vi "Login.vi"() -> ()   [LabVIEW 2020]
uses:
  System.Windows.Forms
  Global_Variable/Global.vi
  <userlib>/_MGI/Menu Building/MenuItemStatusChange/MGI_MenuItemStatusChange.lvclass
panel:
  in  "枚举":enum16{"左工位", "右工位"}(ring)
  in  "菜单":refnum<k24>(container)
  in  "联机模式":enum16{"单机", "追溯"}(ring)
  in  "登陆":bool
  in  "密   码":string
  in  "用户名":string
  out "数据库连接成功":bool
  # "传感器对中台"
  # "数据库状态"
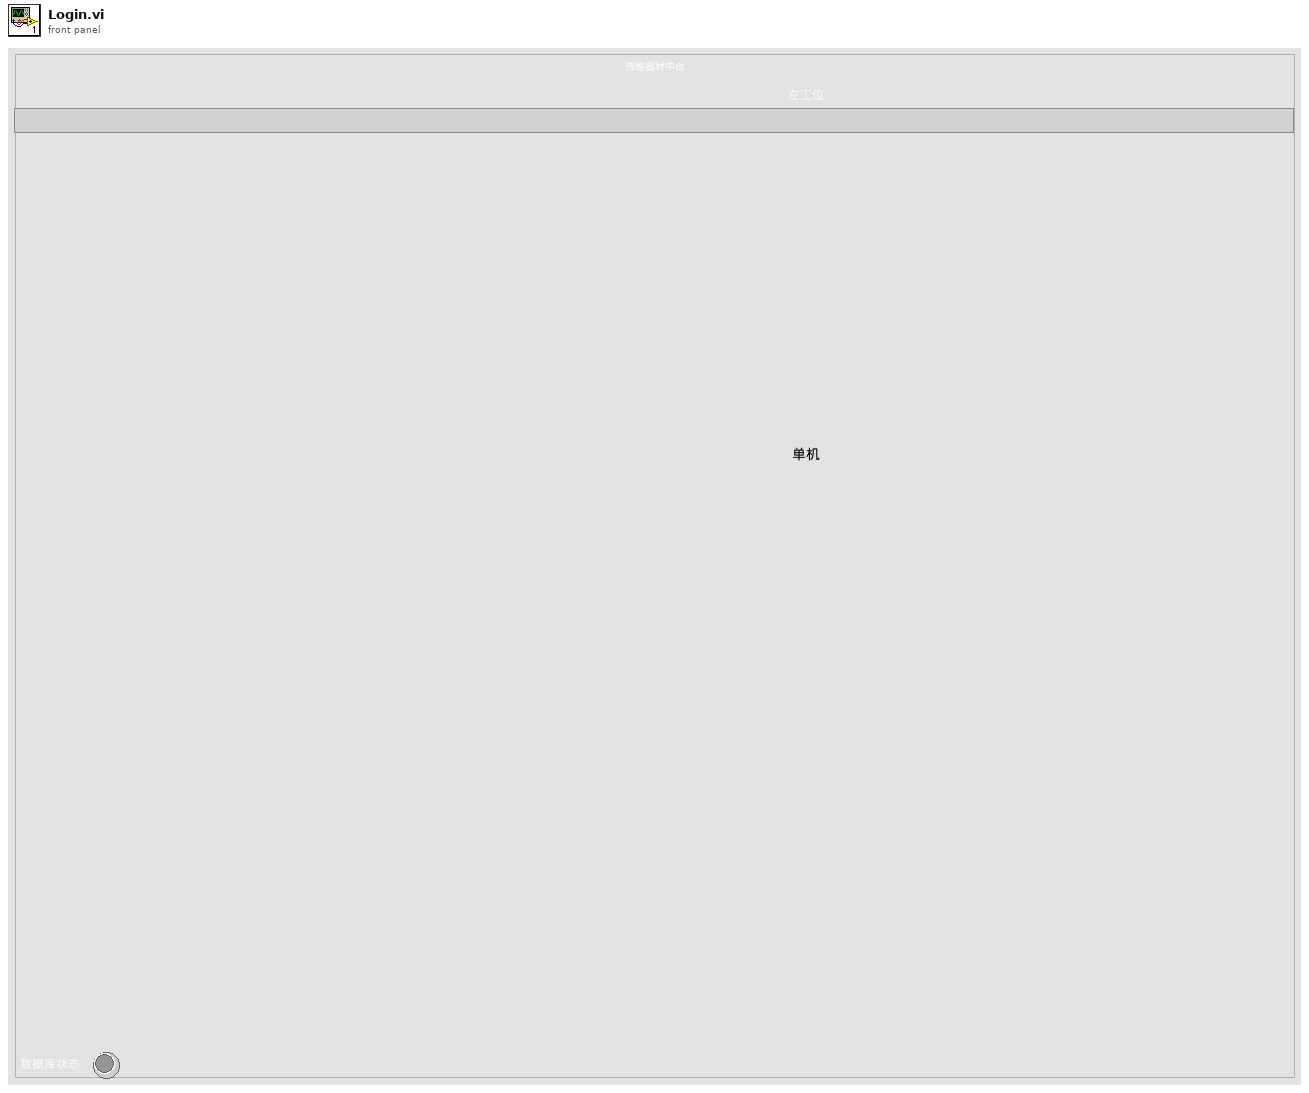
[diagram p1: front panel]
types:
  T1 = enum8{"Enabled", "Disabled", "Disabled and Grayed Out"}
  T2 = enum32{"Invalid", "Standard", "Closed", "Hidden", "Minimized", "Maximized"}
  T3 = cluster{"data[0]":string, "data[1]":string, "data[2]":string, "data[3]":string}
  T4 = typedef "eventvkey.ctl" = enum16{"ASCII", "Enter", "Return", "Shift", "Ctrl", "Alt", "Cmd", "Opt", "Caps", "NumLock", "Clear", "Break", "Up", "Down", "Left", "Right", "Insert", "Delete", "Home", "End", "PageUp", "PageDown", "Escape", "Help", "Pause", "ScrollLock", "F1", "F2", "F3", "F4", "F5", "F6", "F7", "F8", "F9", "F10", "F11", "F12", "F13", "F14", "F15", "F16", "F17", "F18", "F19", "F20", "F21", "F22", "F23", "F24", "Play", "VolumeUp", "VolumeDown", "Mute", "Two Byte Char"}
  T5 = cluster{"用户编号":string, "用户名":string, "用户密码(密文)":string, "用户权限":string}
  T6 = cluster{"操作员编号":string, "操作员姓名":string, "操作员权限":string, "联机模式":enum16{"单机", "追溯"}}
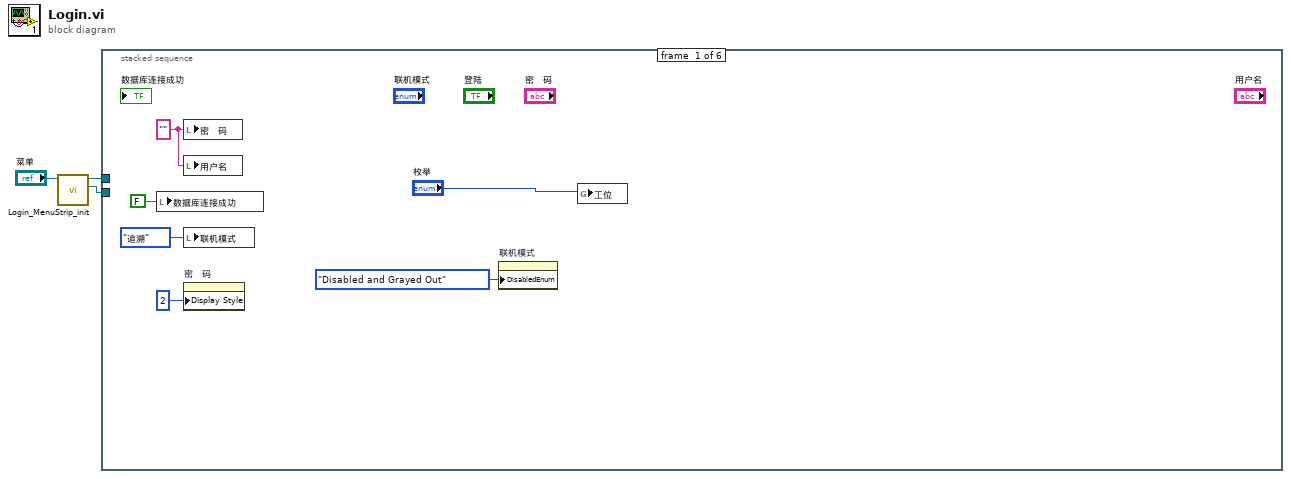
[diagram p0: block diagram]
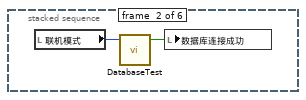
[diagram p2: hidden frame]
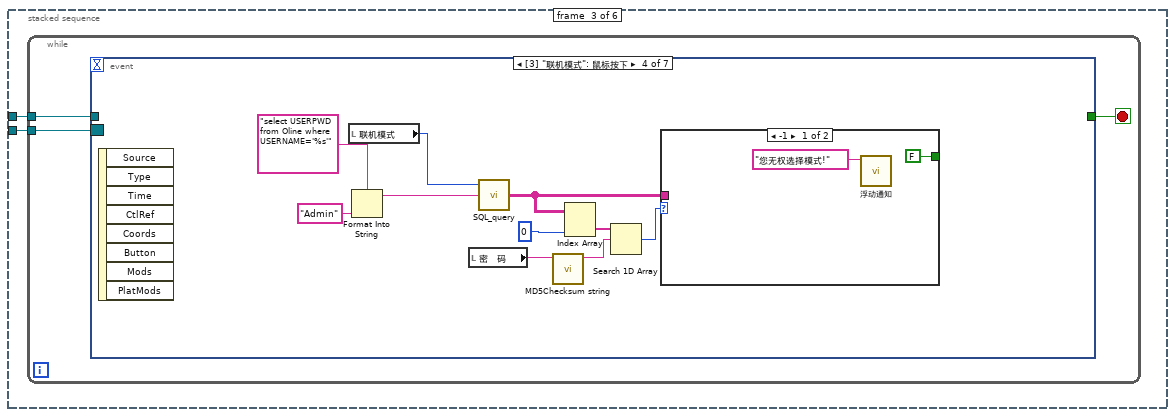
[diagram p3: hidden frame]
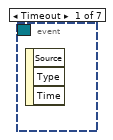
[diagram p4: hidden frame]
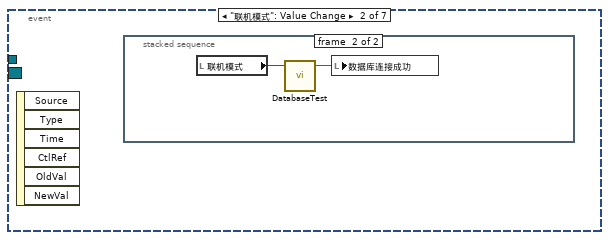
[diagram p5: hidden frame]
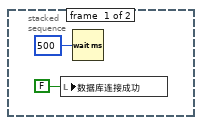
[diagram p6: hidden frame]
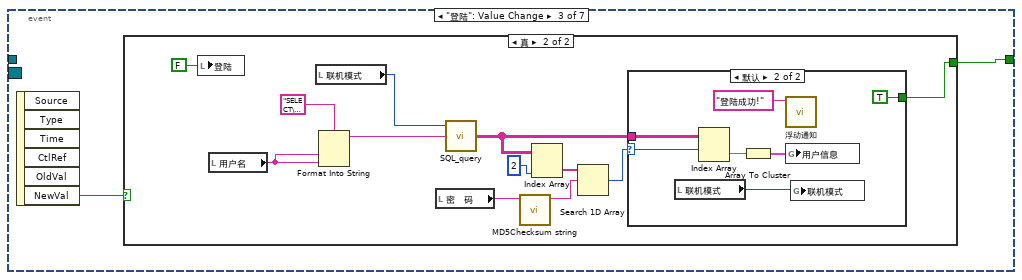
[diagram p7: hidden frame]
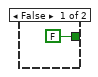
[diagram p8: hidden frame]
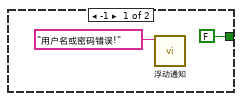
[diagram p9: hidden frame]
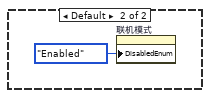
[diagram p10: hidden frame]
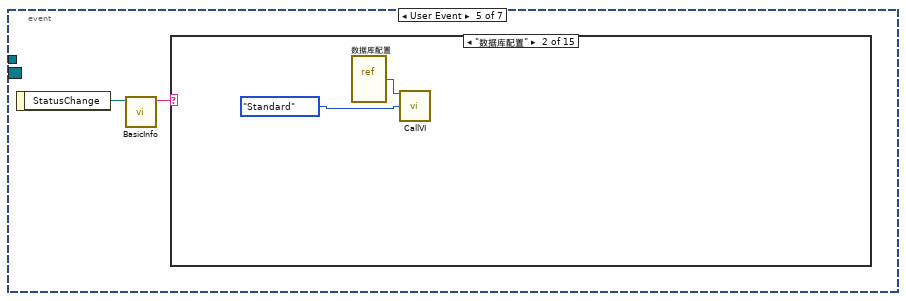
[diagram p11: hidden frame]
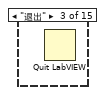
[diagram p13: hidden frame]
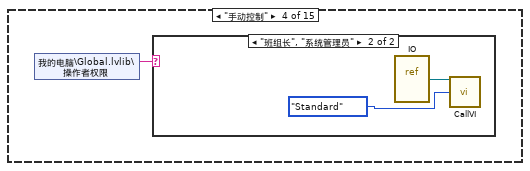
[diagram p14: hidden frame]
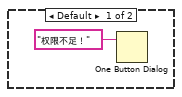
[diagram p15: hidden frame]
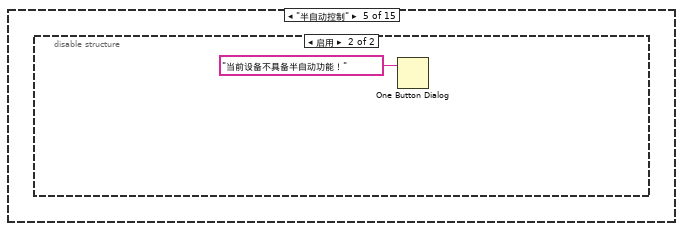
[diagram p16: hidden frame]
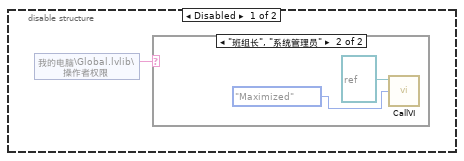
[diagram p17: hidden frame]
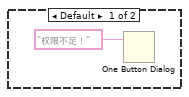
[diagram p18: hidden frame]
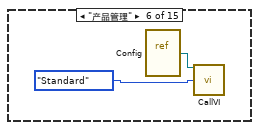
[diagram p19: hidden frame]
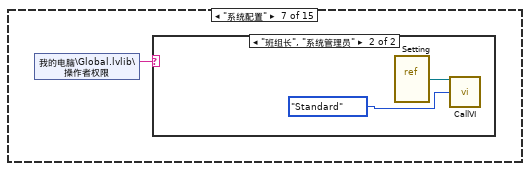
[diagram p20: hidden frame]
diagram:
  n1 = call "Login_MenuStrip_init.vi"("MenuStrip"="菜单") -> ("MenuStrip_Event"=w2:refnum<event-registration>, "Menu out"=w1:refnum<class "MGI_MenuStrip.lvclass">)  [unwired: 9 in]
  n2 = stacked-sequence {
    tunnel: w2 -> [_ _ w13 _ _ _]
    tunnel: w1 -> [_ _ w12 _ _ _]
    frame #0 {
      w8 = ""
      n3 = local write "数据库连接成功"(FALSE ("数据库连接成功")) -> ()
      n4 = local write "密   码"(w8) -> ()
      n5 = local write "用户名"(w8) -> ()
      n6 = local write "联机模式"(enum16{"单机", "追溯"}."追溯" ("联机模式")) -> ()
      n7 = property on="密   码" class="Str"("Display Style"=u32 2 ("显示样式")) -> ()  [unwired: 2 in, 2 out]
      n8 = property on="联机模式" class="Enum (严格)"("DisabledEnum"=T1."Disabled and Grayed Out" ("禁用")) -> ()  [unwired: 2 in, 2 out]
      n9 = global write "Global.vi" "工位"("枚举") -> ()
    }
    frame #1 {
      n10 = local read "联机模式"() -> (w10:enum16{"单机", "追溯"})
      n11 = call "DatabaseTest.vi"("联机模式"=w10) -> ("数据库连接成功"=w11:bool)  [unwired: 3 in, 1 out]
      n12 = local write "数据库连接成功"(w11) -> ()
    }
    frame #2 {
      n13 = while {
        tunnel: w13 -> [w15]
        tunnel: w12 -> [w14]
        stop <- w16 stop-if-true
        n14 = event shown="[3] \"联机模式\": 鼠标按下" {
          selector: w15 -> [_ _ _ _ _ _ _]
          dyn-events: _ -> [_ _ _ _ _ _ _]
          timeout: _ -> [_ _ _ _ _ _ _]
          tunnel: [_ _ w21 _ _ _ TRUE] -> w16
          tunnel: w14 -> [_ _ _ _ _ _ _]
          event Timeout {
            n15 = event-data() -> ()  [unwired: 1 in, 3 out]
          }
          event "联机模式": Value Change {
            n16 = event-data() -> ()  [unwired: 1 in, 6 out]
            n17 = stacked-sequence {
              frame #0 {
                n18 = local write "数据库连接成功"(FALSE ("数据库连接成功")) -> ()
                n19 = Wait (ms)(milliseconds to wait=u32 500 ("等待时间（毫秒）")) -> ()  [unwired: 1 out]
              }
              frame #1 {
                n20 = local read "联机模式"() -> (w19:enum16{"单机", "追溯"})
                n21 = call "DatabaseTest.vi"("联机模式"=w19) -> ("数据库连接成功"=w20:bool)  [unwired: 3 in, 1 out]
                n22 = local write "数据库连接成功"(w20) -> ()
              }
            }
          }
          event "登陆": Value Change {
            n23 = event-data() -> ("NewVal"=w22:bool)  [unwired: 1 in, 5 out]
            n24 = case shown="真" w22 {
              tunnel: [FALSE w26] -> w21
              frame False {
              }
              frame True {
                n25 = local write "登陆"(FALSE ("确定")) -> ()
                n26 = local read "用户名"() -> (w32:string)
                n27 = local read "联机模式"() -> (w24:enum16{"单机", "追溯"})
                n28 = Format Into String(format string="SELECT\ndbo.[User].USER_EMPLOYEE_ID,\ndbo.[User].USER_NAME,\ndbo.[User].USER_PASSWD,\ndbo.[User].USER_PERMIT\n\nFROM\ndbo.[User]\nWHERE\ndbo.[User].USER_NAME = '%s' \nOR\ndbo.[User].USER_EMPLOYEE_ID = '%s'\n" ("格式字符串"), w32, w32) -> (resulting string=w29:string)  [unwired: 2 in, 1 out]
                n29 = local read "密   码"() -> (w33:string)
                n30 = call "SQL_query.vi"("SQL query"=w29, "联机模式"=w24) -> ("data"=w27:string[][])  [unwired: 2 in, 1 out]
                n31 = call <vilib>:"MD5Checksum string.vi"("Message String"=w33) -> ("MD5 message-digest"=w34:string)  [unwired: 10 in]
                n32 = Index Array(array=w27, index (col)=2 ("禁用的索引 (列)")) -> (element=w31:string[])  [unwired: 1 in]
                n33 = Search 1D Array(1D array=w31, element=w34) -> (index of element=w28:i32)  [unwired: 1 in]
                n34 = case shown="默认" w28 {
                  selector: w28 -> [_ w43]
                  tunnel: w27 -> [_ w44]
                  tunnel: [FALSE TRUE] -> w26
                  frame -1 {
                    n35 = call "浮动通知.vi"("通知内容"="用户名或密码错误!") -> ()  [unwired: 11 in]
                  }
                  frame Default {
                    n36 = local read "联机模式"() -> (w38:enum16{"单机", "追溯"})
                    n37 = Index Array(array=w44, index (row)=w43) -> (element=w41:string[])  [unwired: 1 in]
                    n38 = Array To Cluster(array=w41) -> (cluster=w40:T3)
                    n39 = call "浮动通知.vi"("通知内容"="登陆成功!") -> ()  [unwired: 11 in]
                    n40 = global write "Global.vi" "用户信息"(w40) -> ()
                    n41 = global write "Global.vi" "联机模式"(w38) -> ()
                  }
                }
              }
            }
          }
          event "联机模式": Mouse Down {
            n42 = event-data() -> ()  [unwired: 1 in, 8 out]
            n43 = local read "联机模式"() -> (w48:enum16{"单机", "追溯"})
            n44 = Format Into String(format string="select USERPWD from Oline where USERNAME='%s'" ("格式字符串"), "Admin" ("输入 1")) -> (resulting string=w51:string)  [unwired: 2 in, 1 out]
            n45 = local read "密   码"() -> (w53:string)
            n46 = call "SQL_query.vi"("SQL query"=w51, "联机模式"=w48) -> ("data"=w49:string[][])  [unwired: 2 in, 1 out]
            n47 = call <vilib>:"MD5Checksum string.vi"("Message String"=w53) -> ("MD5 message-digest"=w54:string)  [unwired: 10 in]
            n48 = Index Array(array=w49, index (col)=0 ("禁用的索引 (列)")) -> (element=w52:string[])  [unwired: 1 in]
            n49 = Search 1D Array(1D array=w52, element=w54) -> (index of element=w50:i32)  [unwired: 1 in]
            n50 = case shown="-1" w50 {
              tunnel: w49 -> [_ _]
              tunnel: [FALSE _] -> _
              frame -1 {
                n51 = call "浮动通知.vi"("通知内容"="您无权选择模式!") -> ()  [unwired: 11 in]
              }
              frame Default {
                n52 = property on="联机模式" class="Enum (严格)"("DisabledEnum"=T1."Enabled" ("禁用")) -> ()  [unwired: 2 in, 2 out]
              }
            }
          }
          event User Event {
            n53 = event-data() -> ("StatusChange"=w59:refnum<class "MGI_MenuItemStatusChange.lvclass">)  [unwired: 1 in]
            n54 = call <userlib>:"BasicInfo.vi"("MGI_MenuItemStatusChange in"=w59) -> ("Tag"=w58:string)  [unwired: 7 in, 3 out]
            n55 = case shown="\"数据库配置\"" w58 {
              frame "假", Default {
              }
              frame "数据库配置" {
                n56 = vi-ref "数据库配置.vi"() -> (w61:refnum<vi>)
                n57 = call "CallVI.vi"("VI引用"=w61, "状态"=T2."Standard") -> ()  [unwired: 12 in, 2 out]
              }
              frame "退出" {
                n58 = Quit LabVIEW() -> ()  [unwired: 1 in]
              }
              frame "手动控制" {
                n59 = shared-variable "我的电脑\\Global.lvlib\\操作者权限"() -> (w62:string)  [unwired: 1 in, 1 out]
                n60 = case shown="\"班组长\", \"系统管理员\"" w62 {
                  frame Default {
                    n61 = One Button Dialog(message="权限不足！" ("消息")) -> ()  [unwired: 1 in, 1 out]
                  }
                  frame "班组长", "系统管理员" {
                    n62 = vi-ref "IO.vi"() -> (w65:refnum<vi>)
                    n63 = call "CallVI.vi"("VI引用"=w65, "状态"=T2."Standard") -> ()  [unwired: 12 in, 2 out]
                  }
                }
              }
              frame "半自动控制" {
                n64 = disable-structure shown="启用" {
                  frame Disabled {
                    n65 = shared-variable "我的电脑\\Global.lvlib\\操作者权限"() -> (w66:string)  [unwired: 1 in, 1 out]
                    n66 = case shown="\"班组长\", \"系统管理员\"" w66 {
                      frame Default {
                        n67 = One Button Dialog(message="权限不足！" ("消息")) -> ()  [unwired: 1 in, 1 out]
                      }
                      frame "班组长", "系统管理员" {
                        n68 = call "CallVI.vi"("VI引用"=refnum<vi> refnum, "状态"=T2."Maximized") -> ()  [unwired: 12 in, 2 out]
                      }
                    }
                  }
                  frame Enabled {
                    n69 = One Button Dialog(message="当前设备不具备半自动功能！" ("消息")) -> ()  [unwired: 1 in, 1 out]
                  }
                }
              }
              frame "产品管理" {
                n70 = vi-ref "Config.vi"() -> (w72:refnum<vi>)
                n71 = call "CallVI.vi"("VI引用"=w72, "状态"=T2."Standard") -> ()  [unwired: 12 in, 2 out]
              }
              frame "系统配置" {
                n72 = shared-variable "我的电脑\\Global.lvlib\\操作者权限"() -> (w73:string)  [unwired: 1 in, 1 out]
                n73 = case shown="\"班组长\", \"系统管理员\"" w73 {
                  frame Default {
                    n74 = One Button Dialog(message="权限不足！" ("消息")) -> ()  [unwired: 1 in, 1 out]
                  }
                  frame "班组长", "系统管理员" {
                    n75 = vi-ref "Setting.vi"() -> (w76:refnum<vi>)
                    n76 = call "CallVI.vi"("VI引用"=w76, "状态"=T2."Standard") -> ()  [unwired: 12 in, 2 out]
                  }
                }
              }
              frame "用户管理" {
                n77 = shared-variable "我的电脑\\Global.lvlib\\操作者权限"() -> (w77:string)  [unwired: 1 in, 1 out]
                n78 = case shown="\"系统管理员\"" w77 {
                  frame Default {
                    n79 = One Button Dialog(message="权限不足！" ("消息")) -> ()  [unwired: 1 in, 1 out]
                  }
                  frame "系统管理员" {
                    n80 = vi-ref "User_manager.vi"() -> (w80:refnum<vi>)
                    n81 = call "CallVI.vi"("VI引用"=w80, "状态"=T2."Standard") -> ()  [unwired: 12 in, 2 out]
                  }
                }
              }
              frame "编码规则" {
                n82 = shared-variable "我的电脑\\Global.lvlib\\操作者权限"() -> (w81:string)  [unwired: 1 in, 1 out]
                n83 = case shown="\"班组长\", \"工艺管理员\", \"系统管理员\"" w81 {
                  frame Default {
                    n84 = One Button Dialog(message="权限不足！" ("消息")) -> ()  [unwired: 1 in, 1 out]
                  }
                  frame "班组长", "工艺管理员", "系统管理员" {
                    n85 = vi-ref "编码规则设置.vi"() -> (w84:refnum<vi>)
                    n86 = call "CallVI.vi"("VI引用"=w84, "状态"=T2."Standard") -> ()  [unwired: 12 in, 2 out]
                  }
                }
              }
              frame "易损件管理" {
                n87 = vi-ref "易损件管理.vi"() -> (w86:refnum<vi>)
                n88 = call "CallVI.vi"("VI引用"=w86, "状态"=T2."Standard") -> ()  [unwired: 12 in, 2 out]
              }
              frame "物料批次管理" {
                n89 = vi-ref "批次管理.vi"() -> (w88:refnum<vi>)
                n90 = call "CallVI.vi"("VI引用"=w88, "状态"=T2."Standard") -> ()  [unwired: 12 in, 2 out]
              }
              frame "报表" {
                n91 = call "文件对话框"("start path"=path "D:/report", "prompt"="打开报表", "pattern (all files)"="*.doc;*.docx", "pattern label"="Word 文档") -> ("selected path"=w89:path, "error out"=w90:errorcluster)  [unwired: 8 in, 2 out]
                n92 = case shown="无错误" w90 {
                  selector: w90 -> [w96 w98]
                  tunnel: w89 -> [w97 _]
                  frame No Error {
                    w95 = 1 items=["Normal", "Maximize", "Minimize"] ("cpubbs_WindowState")
                    n93 = call "Open_Word.vi"("File Path"=w97, "cpubbs_WindowState"=w95, "错误输入（无错误）"=w96) -> ()  [unwired: 12 in, 1 out]
                  }
                  frame Error {
                    n94 = call <vilib>:"Clear Errors.vi"("error in (no error)"=w98) -> ()  [unwired: 5 in, 2 out]
                  }
                }
              }
              frame "报警信息" {
                n95 = vi-ref "报警信息.vi"() -> (w100:refnum<vi>)
                n96 = call "CallVI.vi"("VI引用"=w100, "状态"=T2."Standard") -> ()  [unwired: 12 in, 2 out]
              }
              frame "关于" {
                n97 = vi-ref "About.vi"() -> (w102:refnum<vi>)
                n98 = call "CallVI.vi"("VI引用"=w102, "状态"=T2."Standard") -> ()  [unwired: 12 in, 2 out]
              }
              frame "操作演示" {
                n99 = call <vilib>:"Application Directory.vi"() -> ("Application Directory"=w105:path)
                n100 = Build Path(base path=w105, name or relative path="操作演示" ("名称或相对路径")) -> (appended path=w104:path)
                n101 = call "自动播放ppt.vi"("路径"=w104) -> ()  [unwired: 10 in, 1 out]
              }
            }
          }
          event Key Down {
            n102 = event-data() -> ("VKey"=w106:T4)  [unwired: 1 in, 9 out]
            n103 = case shown="\"Return\"" w106 {
              frame "ASCII", Default {
              }
              frame "Return" {
                n104 = property on="登陆" class="Bool (严格)"("Val(Sgnl)"=TRUE ("值(信号)")) -> ()  [unwired: 2 in, 2 out]
              }
            }
          }
          event Panel Close {
            n105 = event-data() -> ()  [unwired: 1 in, 4 out]
            n106 = Quit LabVIEW() -> ()  [unwired: 1 in]
          }
        }
      }
    }
    frame #3 {
      n107 = global read "Global.vi" "用户信息"() -> (w115:T5)
      n108 = Unbundle By Name(w115) -> ("用户编号"=w110:string, "用户名"=w111:string, "用户权限"=w112:string)  [unwired: 1 out]
      n109 = local read "联机模式"() -> (w109:enum16{"单机", "追溯"})
      n110 = call "Get_Device_ID.vi"() -> ("Device_ID"=w117:string)  [unwired: 10 in, 1 out]
      n111 = global write "追溯Global.vi" "DEVICE_ID"(w117) -> ()
      n112 = global read "用户信息.vi" "用户信息"() -> (w114:T6)
      n113 = call "Get_USER_ID.vi"("USER_EMPLOYEE_ID"=w110) -> ("USER_ID"=w116:string)  [unwired: 9 in, 1 out]
      n114 = Bundle By Name(cluster=w114, "操作员编号"=w110, "操作员姓名"=w111, "操作员权限"=w112, "联机模式"=w109) -> (w113:T6)
      n115 = global write "追溯Global.vi" "USER_ID"(w116) -> ()
      n116 = global write "用户信息.vi" "用户信息"(w113) -> ()
    }
    frame #4 {
      n117 = vi-ref "Main.vi"() -> (w119:refnum<vi>)
      n118 = call "CallVI.vi"("VI引用"=w119, "状态"=T2."Maximized") -> ()  [unwired: 12 in, 2 out]
    }
    frame #5 {
      n119 = control-ref of="本VI"() -> (w120:refnum<vi>)
      n120 = invoke class="VI" method="FP.Close"(reference=w120) -> (reference out=w121:refnum<vi>, error out=w122:errorcluster)  [unwired: 2 in, 1 out]
      n121 = Close Reference(reference=w121, error in (no error)=w122) -> ()  [unwired: 1 out]
    }
  }
